vi "UHR-Fleezers Control (host) - 10.5.vi"() -> ()   [LabVIEW 2010] (continued)
          tunnel: [w3296 w3297] -> w3263
          frame False {
          }
          frame True {
            n566 = Array Subset(array=w3302, index (row)=0 ("index"), length (row)=4 ("length"), index (col)=0 ("index"), length (col)=1 ("length")) -> (w3297:T44)
          }
        }
        n567 = feedback-in #9(w3263) -> ()
        n568 = Split 1D Array(array=w3277, index=2) -> (first subarray=→"FFT 1":cluster{"f0":dbl, "df":dbl, "magnitude":dbl[]}[], second subarray=→"FFT 2":cluster{"f0":dbl, "df":dbl, "magnitude":dbl[]}[])
      }
    }
    n569 = Index Array(array=w1002, index=1) -> (element=w1010:waveform(dbl))
    n570 = case "For displaying the high resolution display (no downsampling)" shown="True" w1075 {
      tunnel: w1029 -> [_ w1535]
      frame False {
      }
      frame True {
        n571 = Index Array(array=w1535, index="High Res. Display") -> (element=w1536:waveform(dbl))
        n572 = call <vilib>:"Std Deviation and Variance.vi"("X"=w1536) -> ("mean"=w1543:dbl, "standard deviation"=w1548:dbl)  [unwired: 1 in, 1 out]
        "Mean Intensity" <- w1543
        "Sigma" <- w1548
        n573 = Subtract(x=w1536, y=w1543) -> (x-y=w1542:waveform(dbl))
        n574 = Select(t=w1542, s="Subtract mean", f=w1536) -> (s? t:f=→"1 Channel":waveform(dbl))
        n575 = Divide(x=w1548, y=w1543) -> (x/y=→"Sigma/Mean":dbl)
        n576 = feedback #10(1) -> (w1537:i32)
        n577 = Greater Or Equal?(x=w1537, y="Slow mean N ave.") -> (x >= y?=w1550:bool)
        n578 = Increment(x=w1537) -> (x+1=w1552:i32)
        n579 = Select(t=1, s=w1550, f=w1552) -> (s? t:f=w1539:i32)
        n580 = feedback-in #10(w1539) -> ()
        n581 = feedback #11() -> (w1540:waveform(dbl))  [unwired: 1 out]
        n582 = case shown="Default" w1537 {
          tunnel: [w1555 w1558] -> w1541
          tunnel: w1540 -> [w1557 _]
          tunnel: w1536 -> [w1556 w1558]
          frame Default {
            n583 = call-poly <vilib>:"Append Waveforms.vi"("waveform B"=w1556, "waveform A"=w1557) -> ("waveform out"=w1555:waveform(dbl))  [unwired: 1 in, 8 out]
          }
          frame 1 {
          }
        }
        n584 = feedback-in #11(w1541) -> ()
        n585 = case shown="True" w1550 {
          tunnel: w1541 -> [_ w1554]
          frame False {
          }
          frame True {
            n586 = call <vilib>:"Mean.vi"("X"=w1554) -> ("mean"=→"Slow mean":dbl)  [unwired: 1 out]
          }
        }
      }
    }
    n587 = case "For plotting results of scanning MCL" shown="True" w1152 {
      tunnel: w1151 -> [_ w2066]
      tunnel: w1068 -> [_ w2162]
      tunnel: w1160 -> [_ _]
      tunnel: w1029 -> [_ w2136]
      tunnel: w1004 -> [_ w2067]
      tunnel: w1003 -> [_ w2040]
      frame False {
      }
      frame True {
        w2047 = u32 0 items=["Horizontal", "Vertical", "Central", "1st Diagonal", "2nd Diagonal"] ("Type of Symmetry")
        w2075 = u32 0 items=["Horizontal", "Vertical", "Central", "1st Diagonal", "2nd Diagonal"] ("Type of Symmetry")
        w2078 = u32 0 items=["Horizontal", "Vertical", "Central", "1st Diagonal", "2nd Diagonal"] ("Type of Symmetry")
        w2107 = u32 0 items=["Horizontal", "Vertical", "Central", "1st Diagonal", "2nd Diagonal"] ("Type of Symmetry")
        n588 = Index Array(array=w2136, index=10) -> (element=w2142:waveform(dbl))
        n589 = Index Array(array=w2136, index=11) -> (element=w2139:waveform(dbl))
        n590 = local read "Cycles/step (MCL)"() -> (w2092:u64)
        n591 = Index Array(array=w2136, index="Channel") -> (element=w2138:waveform(dbl))
        n592 = Unbundle(w2040) -> ("New Image"=w2039:T2, "New Image"=w2038:T2, "New Image"=w2037:T2, "New Image"=w2036:T2)
        n593 = Unbundle By Name(w2142) -> ("Y"=w2094:dbl[])
        n594 = Unbundle By Name(w2139) -> ("Y"=w2096:dbl[])
        n595 = Unbundle By Name(w2138) -> ("Y"=w2101:dbl[])
        n596 = call "downsample 1D array - double.vi"("Ave N"=w2092, "Array In"=w2094) -> ("Array Out"=w2093:dbl[])  [unwired: 1 out]
        n597 = call "downsample 1D array - double.vi"("Ave N"=w2092, "Array In"=w2096) -> ("Array Out"=w2095:dbl[])  [unwired: 1 out]
        n598 = call "downsample 1D array - double.vi"("Ave N"=w2092, "Array In"=w2101) -> ("Array Out"=w2100:dbl[])  [unwired: 1 out]
        n599 = feedback #12(w2162) -> (w2163:dbl[])
        n600 = Build Array (concatenate)(w2163, w2162) -> (w2144:dbl[])
        n601 = feedback #13(w2067) -> (w2069:dbl[])
        n602 = Build Array (concatenate)(w2069, w2067) -> (w2068:dbl[])
        n603 = local read "Scan steps (MCL)"() -> (w2049:u64)
        n604 = Select(t=w2162, s=w2066, f=w2144) -> (s? t:f=w2148:dbl[])
        n605 = feedback-in #12(w2148) -> ()
        n606 = Select(t=w2067, s=w2066, f=w2068) -> (s? t:f=w2050:dbl[])
        n607 = feedback-in #13(w2050) -> ()
        n608 = local read "Scan lines (y)"() -> (w2035:u64)
        n609 = local read "N APD Samp/step"() -> (w2051:dbl)
        n610 = feedback #14(w2093) -> (w2150:dbl[])
        n611 = Build Array (concatenate)(w2150, w2093) -> (w2141:dbl[])
        n612 = feedback #15(w2100) -> (w2160:dbl[])
        n613 = Build Array (concatenate)(w2160, w2100) -> (w2159:dbl[])
        n614 = feedback #16(w2095) -> (w2152:dbl[])
        n615 = Build Array (concatenate)(w2152, w2095) -> (w2153:dbl[])
        n616 = Select(t=w2093, s=w2066, f=w2141) -> (s? t:f=w2097:dbl[])
        n617 = feedback-in #14(w2097) -> ()
        n618 = Select(t=w2100, s=w2066, f=w2159) -> (s? t:f=w2099:dbl[])
        n619 = feedback-in #15(w2099) -> ()
        n620 = Select(t=w2095, s=w2066, f=w2153) -> (s? t:f=w2098:dbl[])
        n621 = feedback-in #16(w2098) -> ()
        n622 = Multiply(x=w2049, y=u64 2) -> (x*y=w2034:u64)
        n623 = call "integrate 1D array interval - double.vi"("Ave N"=w2051, "Array In"=w2050) -> ("Array Out"=w2062:dbl[])  [unwired: 1 out]
        n624 = call "integrate 1D array interval - double.vi"("Ave N"=w2051, "Array In"=w2148) -> ("Array Out"=w2147:dbl[])  [unwired: 1 out]
        n625 = Array Size(array=w2062) -> (size(s)=w2063:i32)
        n626 = Array Size(array=w2147) -> (size(s)=w2149:i32)
        n627 = Multiply(x=w2035, y=w2034) -> (x*y=w2065:u64)
        n628 = Multiply(x=w2035, y=w2034) -> (x*y=w2157:u64)
        n629 = call <vilib>:"Mean.vi"("X"=w2097) -> ("mean"=w2081:dbl)  [unwired: 1 out]
        n630 = Subtract(x=w2065, y=w2063) -> (x-y=w2056:u64)
        n631 = call <vilib>:"Mean.vi"("X"=w2099) -> ("mean"=w2086:dbl)  [unwired: 1 out]
        n632 = call <vilib>:"Mean.vi"("X"=w2098) -> ("mean"=w2084:dbl)  [unwired: 1 out]
        n633 = call <vilib>:"Mean.vi"("X"=w2062) -> ("mean"=w2053:dbl)  [unwired: 1 out]
        n634 = Subtract(x=w2157, y=w2149) -> (x-y=w2091:u64)
        n635 = call <vilib>:"Mean.vi"("X"=w2147) -> ("mean"=w2088:dbl)  [unwired: 1 out]
        n636 = Initialize Array(1.0 ("element"), w2056) -> (w2052:dbl[])
        n637 = Initialize Array(1.0 ("element"), w2091) -> (w2082:dbl[])
        n638 = Multiply(x=w2052, y=w2053) -> (x*y=w2054:dbl[])
        n639 = Multiply(x=w2082, y=w2084) -> (x*y=w2085:dbl[])
        n640 = Multiply(x=w2082, y=w2086) -> (x*y=w2087:dbl[])
        n641 = Multiply(x=w2082, y=w2081) -> (x*y=w2083:dbl[])
        n642 = Multiply(x=w2082, y=w2088) -> (x*y=w2089:dbl[])
        n643 = Build Array (concatenate)(w2097, w2083) -> (w2151:dbl[])
        n644 = Build Array (concatenate)(w2099, w2087) -> (w2155:dbl[])
        n645 = Build Array (concatenate)(w2098, w2085) -> (w2154:dbl[])
        n646 = Build Array (concatenate)(w2062, w2054) -> (w2064:dbl[])
        n647 = Build Array (concatenate)(w2147, w2089) -> (w2156:dbl[])
        n648 = Reshape Array(w2151, w2035, w2034) -> (w2117:dbl[][])
        n649 = Reshape Array(w2064, w2035, w2034) -> (w2060:dbl[][])
        n650 = Reshape Array(w2155, w2035, w2034) -> (w2109:dbl[][])
        n651 = Reshape Array(w2154, w2035, w2034) -> (w2124:dbl[][])
        n652 = Reshape Array(w2156, w2035, w2034) -> (w2134:dbl[][])
        n653 = Array Subset(array=w2124, index (col)=0 ("index"), length (col)=w2049) -> (w2129:dbl[][])  [unwired: 2 in]
        n654 = Array Subset(array=w2124, index (col)=w2049) -> (w2127:dbl[][])  [unwired: 3 in]
        n655 = Array Subset(array=w2109, index (col)=0 ("index"), length (col)=w2049) -> (w2115:dbl[][])  [unwired: 2 in]
        n656 = Array Subset(array=w2109, index (col)=w2049) -> (w2113:dbl[][])  [unwired: 3 in]
        n657 = Array Subset(array=w2060, index (col)=0 ("index"), length (col)=w2049) -> (w2059:dbl[][])  [unwired: 2 in]
        n658 = Array Subset(array=w2060, index (col)=w2049) -> (w2057:dbl[][])  [unwired: 3 in]
        n659 = Array Subset(array=w2134, index (col)=0 ("index"), length (col)=w2049) -> (w2133:dbl[][])  [unwired: 2 in]
        n660 = Array Subset(array=w2134, index (col)=w2049) -> (w2131:dbl[][])  [unwired: 3 in]
        n661 = Array Subset(array=w2117, index (col)=0 ("index"), length (col)=w2049) -> (w2122:dbl[][])  [unwired: 2 in]
        n662 = Array Subset(array=w2117, index (col)=w2049) -> (w2120:dbl[][])  [unwired: 3 in]
        n663 = for {
          tunnel: w2129 -> [w2171] mode=indexing
          tunnel: [w2170] -> w2128 mode=indexing
          workers-P: _ -> [_]
          n664 = Reverse 1D Array(array=w2171) -> (reversed array=w2170:dbl[])
        }
        n665 = for {
          tunnel: w2115 -> [w2167] mode=indexing
          tunnel: [w2166] -> w2114 mode=indexing
          workers-P: _ -> [_]
          n666 = Reverse 1D Array(array=w2167) -> (reversed array=w2166:dbl[])
        }
        n667 = for {
          tunnel: w2059 -> [w2165] mode=indexing
          tunnel: [w2164] -> w2058 mode=indexing
          workers-P: _ -> [_]
          n668 = Reverse 1D Array(array=w2165) -> (reversed array=w2164:dbl[])
        }
        n669 = for {
          tunnel: w2133 -> [w2173] mode=indexing
          tunnel: [w2172] -> w2132 mode=indexing
          workers-P: _ -> [_]
          n670 = Reverse 1D Array(array=w2173) -> (reversed array=w2172:dbl[])
        }
        n671 = for {
          tunnel: w2122 -> [w2169] mode=indexing
          tunnel: [w2168] -> w2121 mode=indexing
          workers-P: _ -> [_]
          n672 = Reverse 1D Array(array=w2169) -> (reversed array=w2168:dbl[])
        }
        n673 = Index Array(array=w2134, index (row)=0) -> (element=→"Waveform Graph":dbl[])  [unwired: 1 in]
        n674 = Add(x=w2128, y=w2127) -> (x+y=w2126:dbl[][])
        n675 = Add(x=w2114, y=w2113) -> (x+y=w2112:dbl[][])
        n676 = Add(x=w2058, y=w2057) -> (x+y=w2042:dbl[][])
        n677 = Add(x=w2132, y=w2131) -> (x+y=w2106:dbl[][])
        n678 = Add(x=w2121, y=w2120) -> (x+y=w2119:dbl[][])
        n679 = Divide(x=w2112, y=2) -> (x/y=w2110:dbl[][])
        n680 = Divide(x=w2126, y=2) -> (x/y=w2071:dbl[][])
        n681 = Divide(x=w2119, y=2) -> (x/y=w2073:dbl[][])
        n682 = To Single Precision Float(number=w2106) -> (single precision float=w2105:sgl[][])
        n683 = Transpose 2D Array(2D array=w2110) -> (transposed array=→"Data map":dbl[][])
        n684 = To Single Precision Float(number=w2042) -> (single precision float=w2046:sgl[][])
        n685 = To Single Precision Float(number=w2071) -> (single precision float=w2077:sgl[][])
        n686 = To Single Precision Float(number=w2073) -> (single precision float=w2074:sgl[][])
        n687 = call "IMAQ ArrayToImage"("Image Pixels (Float)"=w2105, "Image"=w2039) -> ("Image Out"=w2108:T2)  [unwired: 8 in, 1 out]
        n688 = call "IMAQ ArrayToImage"("Image Pixels (Float)"=w2046, "Image"=w2038) -> ("Image Out"=w2048:T2)  [unwired: 8 in, 1 out]
        n689 = call "IMAQ ArrayToImage"("Image Pixels (Float)"=w2077, "Image"=w2037) -> ("Image Out"=w2079:T2)  [unwired: 8 in, 1 out]
        n690 = call "IMAQ ArrayToImage"("Image Pixels (Float)"=w2074, "Image"=w2036) -> ("Image Out"=w2076:T2)  [unwired: 8 in, 1 out]
        n691 = call "IMAQ Symmetry"("Type of Symmetry"=w2107, "Image Src"=w2108) -> ("Image Dst Out"=w2103:T2)  [unwired: 3 in, 1 out]
        n692 = call "IMAQ Symmetry"("Type of Symmetry"=w2047, "Image Src"=w2048) -> ("Image Dst Out"=w2044:T2)  [unwired: 3 in, 1 out]
        n693 = call "IMAQ Symmetry"("Type of Symmetry"=w2078, "Image Src"=w2079) -> ("Image Dst Out"=→"Detection Laser X":T2)  [unwired: 3 in, 1 out]
        n694 = call "IMAQ Symmetry"("Type of Symmetry"=w2075, "Image Src"=w2076) -> ("Image Dst Out"=→"Detection Laser Y":T2)  [unwired: 3 in, 1 out]
        n695 = call "IMAQ Set Simple Calibration"("Calibration Axis Info"=T31 {"Origin Pixel"={"X"=0.0, "Y"=0.0}, "Angle Relative to Horizontal (deg)"=0.0, "Axis Reference"=0}, "Grid Descriptor"=T32 {"X Step"=0.3, "Y Step"=0.3, "Unit"=enum."Undefined"}, "Image"=w2103) -> ("Calibrated Image"=→"APD 1":T2)  [unwired: 7 in, 1 out]
        n696 = call "IMAQ Set Simple Calibration"("Calibration Axis Info"=T31 {"Origin Pixel"={"X"=0.0, "Y"=0.0}, "Angle Relative to Horizontal (deg)"=0.0, "Axis Reference"=0}, "Grid Descriptor"=T32 {"X Step"=0.3, "Y Step"=0.3, "Unit"=enum."Undefined"}, "Image"=w2044) -> ("Calibrated Image"=→"APD 2":T2)  [unwired: 7 in, 1 out]
      }
    }
    n697 = Subtract(x=w1010, y="APD 2 Offset") -> (x-y=w1007:waveform(dbl))
    n698 = Subtract(x=w1012, y="APD 1 Offset") -> (x-y=w1008:waveform(dbl))
    n699 = Index Array(array=w1027, index=3) -> (element=w1096:waveform(dbl))
    n700 = Index Array(array=w1027, index=6) -> (element=w1093:waveform(dbl))
    n701 = Build Array(w1008, w1007) -> (→"APD Chart":waveform(dbl)[])
    n702 = Array Size(array=w1085) -> (size(s)=w1140:i32)
    n703 = call <vilib>:"Std Deviation and Variance.vi"("X"=w1020) -> ("standard deviation"=w1019:dbl)  [unwired: 1 in, 2 out]
    n704 = Add Array Elements(numeric array=w1020) -> (sum=w1022:u32)
    n705 = Add Array Elements(numeric array=w1085) -> (sum=w1150:u32)
    n706 = call <vilib>:"Std Deviation and Variance.vi"("X"=w1085) -> ("standard deviation"=w1084:dbl)  [unwired: 1 in, 2 out]
    n707 = Divide(x="T1 offset_x (mV)", y=1000.0) -> (x/y=w1097:dbl)
    n708 = Divide(x=w1019, y=w1018) -> (x/y=w1015:dbl)
    "Rate sigma (Hz) 2" <- w1015
    n709 = Multiply(x=w1018, y=w1140) -> (x*y=w1021:dbl)
    "Int. Time (s)" <- w1021
    n710 = Divide(x=w1022, y=w1021) -> (x/y=w1016:dbl)
    "APD 2 Rate (Hz)" <- w1016
    n711 = Divide(x=w1150, y=w1021) -> (x/y=w1082:dbl)
    "APD 1 Rate (Hz)" <- w1082
    n712 = Divide(x=w1084, y=w1018) -> (x/y=w1083:dbl)
    "Rate sigma (Hz)" <- w1083
    n713 = Divide(x=w1015, y=w1016) -> (x/y=→"Sigma/Mean 2":dbl)
    n714 = Divide(x=w1083, y=w1082) -> (x/y=→"Sigma/Mean":dbl)
    n715 = Divide(x="T2 offset_x (mV)", y=1000.0) -> (x/y=w1095:dbl)
    n716 = case shown="2" "Calibration" {
      tunnel: "T1 alpha_x (nm/V)" -> [_ w2002 w2023]
      tunnel: "T1 kappa_x (pN/nm)" -> [_ _ w2013]
      tunnel: "T2 alpha_x (nm/V)" -> [_ w2001 w2021]
      tunnel: "T2 kappa_x (pN/nm)" -> [_ _ w2014]
      tunnel: w1096 -> [w1984 w1999 w2019]
      tunnel: w1093 -> [w1983 w1997 w2017]
      tunnel: [w1984 w1996 w2016] -> w1126
      tunnel: [w1983 w1995 w2015] -> w1125
      tunnel: ["T1 X (V)" ("Label.Text") "T1 X (nm)" ("Label.Text") "T1 X (pN)" ("Label.Text")] -> w1114
      tunnel: ["T2 X (V)" ("Label.Text") "T2 X (nm)" ("Label.Text") "T2 X (pN)" ("Label.Text")] -> w1113
      tunnel: ["Position (V)" ("Label.Text") "Position (nm)" ("Label.Text") "Force (pN)" ("Label.Text")] -> w1115
      tunnel: w1095 -> [_ w1987 w2006]
      tunnel: w1097 -> [_ w1990 w2008]
      tunnel: ["Mean (V)" ("Label.Text") "Mean (nm)" ("Label.Text") "Mean (pN)" ("Label.Text")] -> w1110
      tunnel: ["Difference (V)" ("Label.Text") "Difference (nm)" ("Label.Text") "Difference (pN)" ("Label.Text")] -> w1035
      frame 0, Default {
      }
      frame 1 {
        # "position"
        n717 = Unbundle By Name(w1999) -> ("Y"=w2003:dbl[])
        n718 = Unbundle By Name(w1997) -> ("Y"=w1988:dbl[])
        n719 = Subtract(x=w2003, y=w1990) -> (x-y=w1991:dbl[])
        n720 = Subtract(x=w1988, y=w1987) -> (x-y=w1989:dbl[])
        n721 = Multiply(x=w1989, y=w2001) -> (x*y=w1998:dbl[])
        n722 = Multiply(x=w2002, y=w1991) -> (x*y=w2000:dbl[])
        n723 = Bundle By Name(cluster=w1997, "Y"=w1998) -> (w1995:waveform(dbl))
        n724 = Bundle By Name(cluster=w1999, "Y"=w2000) -> (w1996:waveform(dbl))
      }
      frame 2 {
        # "force"
        n725 = Unbundle By Name(w2019) -> ("Y"=w2024:dbl[])
        n726 = Unbundle By Name(w2017) -> ("Y"=w2022:dbl[])
        n727 = Subtract(x=w2022, y=w2006) -> (x-y=w2007:dbl[])
        n728 = Subtract(x=w2024, y=w2008) -> (x-y=w2009:dbl[])
        n729 = Compound Arithmetic op=MULTIPLY(w2007, w2021, w2014) -> (w2018:dbl[])
        n730 = Compound Arithmetic op=MULTIPLY(w2013, w2023, w2009) -> (w2020:dbl[])
        n731 = Bundle By Name(cluster=w2017, "Y"=w2018) -> (w2015:waveform(dbl))
        n732 = Bundle By Name(cluster=w2019, "Y"=w2020) -> (w2016:waveform(dbl))
      }
    }
    n733 = feedback-in #17("Calibration") -> ()
    n734 = feedback #17(u16 1 ("Calibration")) -> (w1117:u16)
    n735 = Not Equal?(x=w1117, y="Calibration") -> (x != y?=w1073:bool)
    n736 = Unbundle By Name(w1096) -> ("Y"=w1099:dbl[])
    n737 = Unbundle By Name(w1093) -> ("Y"=w1102:dbl[])
    n738 = Subtract(x=w1099, y=w1097) -> (x-y=w1100:dbl[])
    n739 = Subtract(x=w1102, y=w1095) -> (x-y=w1101:dbl[])
    n740 = Multiply(x=w1101, y="T2 alpha_x (nm/V)") -> (x*y=w1092:dbl[])
    n741 = Multiply(x="T1 alpha_x (nm/V)", y=w1100) -> (x*y=w1091:dbl[])
    n742 = Multiply(x=w1125, y=-1.0) -> (x*y=w1104:waveform(dbl))
    n743 = case shown="True" "Read Lateness and Rel Phase" {
      tunnel: w926 -> [w1559 w1581]
      tunnel: w925 -> [w1560 w1580]
      tunnel: [w1559 w1579] -> w1088
      tunnel: [w1560 w1578] -> w1087
      frame False {
      }
      frame True {
        n744 = xnode "Read/Write Control"("FPGA VI Reference In"=w1581, "error in"=w1580) -> ("FPGA VI Reference Out"=w1579:T20, "error out"=w1578:errorcluster, "GI Relative phase"=→"GI relative phase":i16, "Relative phase"=→"Relative phase (AI1)":i16, "AI Late Counter"=→"Late Counter (AI1)":u16, "GI Late Counter"=→"GI Late Counter":u16, "MCL Late Counter"=→"MCL Late Counter":u16, "MCL Relative Phase"=→"Relative Phase (MCL)":i16, "APD Acq Relative Phase"=→"APD Acq Relative Phase":i16, "APD 1 Gate Relative Phase"=→"APD 1 Gate Relative Phase":i16, "APD 2 Gate Relative Phase"=→"APD 2 Gate Relative Phase":i16, "APD Acq Late Counter"=→"APD Acq Late Counter":u16, "APD 1 Gate Late Counter"=→"APD 1 Gate Late Counter":u16, "APD 2 Gate Late Counter"=→"APD 2 Gate Late Counter":u16, "Green FB Relative Phase"=→"Relative phase (Green FB)":i16, "GI Relative phase 2"=→"GI relative phase 2":i16, "GI Late Counter 2"=→"GI Late Counter 2":u16, "Trap Pos FIFO Timeout"=→"Trap Pos FIFO Timeout":u16, "Trap AI FIFO Timeout"=→"Trap AI FIFO Timeout":u16)
      }
    }
    n745 = Subtract(x=w1092, y=w1091) -> (x-y=w1090:dbl[])
    n746 = Unbundle By Name(w1125) -> ("Y"=w1060:dbl[])
    n747 = Unbundle By Name(w1126) -> ("Y"=w1061:dbl[])
    n748 = Build Array(w1126, w1104) -> (→"Force":waveform(dbl)[])
    n749 = Subtract(x=w1090, y="Offset (nm)") -> (x-y=w1058:dbl[])
    n750 = call <vilib>:"Mean.vi"("X"=w1060) -> ("mean"=w1039:dbl)  [unwired: 1 out]
    "T2 X" <- w1039
    n751 = Absolute Value(x=w1061) -> (abs(x)=w1062:dbl[])
    n752 = Absolute Value(x=w1060) -> (abs(x)=w1063:dbl[])
    n753 = call <vilib>:"Mean.vi"("X"=w1061) -> ("mean"=w1040:dbl)  [unwired: 1 out]
    "T1 X" <- w1040
    n754 = Add(x=w1062, y=w1063) -> (x+y=w1064:dbl[])
    n755 = Bundle By Name(cluster=w1096, "Y"=w1058) -> (w1026:waveform(dbl))
    "Bead Separation" <- w1026
    n756 = Divide(x=w1064, y=2.0) -> (x/y=→"Vec Mean of T1 T2":dbl[])
    n757 = case shown="True" w1073 {
      tunnel: w1115 -> [_ w1977]
      tunnel: w1114 -> [_ w1976]
      tunnel: w1113 -> [_ w1975]
      tunnel: w1110 -> [_ w1974]
      tunnel: w1035 -> [_ w1973]
      frame False {
      }
      frame True {
        n758 = property on="Force" class="WFChart (strict)"("YScale.NameLbl.Text"=w1977) -> ()  [unwired: 2 in, 2 out]
        n759 = property on="T2 X" class="DigNum (strict)"("Caption.Text"=w1975) -> ()  [unwired: 2 in, 2 out]
        n760 = property on="T1 X" class="DigNum (strict)"("Caption.Text"=w1976) -> ()  [unwired: 2 in, 2 out]
        n761 = property on="Mean" class="DigNum (strict)"("Caption.Text"=w1974) -> ()  [unwired: 2 in, 2 out]
        n762 = property on="Difference" class="DigNum (strict)"("Caption.Text"=w1973) -> ()  [unwired: 2 in, 2 out]
      }
    }
    n763 = local read "Tether"() -> (w1067:bool)
    n764 = Absolute Value(x=w1040) -> (abs(x)=w1037:dbl)
    n765 = Absolute Value(x=w1039) -> (abs(x)=w1036:dbl)
    n766 = Add(x=w1037, y=w1036) -> (x+y=w1112:dbl)
    n767 = Subtract(x=w1037, y=w1036) -> (x-y=→"Difference":dbl)
    n768 = feedback #18(w1058) -> (w1057:dbl[])
    n769 = Divide(x=w1112, y=2.0) -> (x/y=w1066:dbl)
    "Mean" <- w1066
    n770 = case shown="True" w1067 {
      tunnel: w1066 -> [_ w1518]
      frame False {
      }
      frame True {
        n771 = Greater?(x="Lost Tether Alarm Threshold (pN)", y=w1518) -> (0:w1516:bool)
        n772 = case shown="True" w1516 {
          frame False {
          }
          frame True {
            n773 = flat-sequence {
              frame #0 {
                # "stop only if saving"
                n774 = local read "Saving..."() -> (w1531:bool)
                n775 = And(x=w1531, y="TA Cancel Save?") -> (x .and. y?=w1530:bool)
                n776 = local write "Stop Saving"(w1530) -> ()
              }
              frame #1 {
                n777 = case shown="True" "TA Green Off?" {
                  frame False {
                  }
                  frame True {
                    w1534 = FALSE ("Fl. Triggered...")
                    n778 = local write "Fl. Triggered..."(w1534) -> ()
                    n779 = property on="Green Laser ON/Interlacing" class="Bool (strict)"("Val(Sgnl)"=w1534) -> ()  [unwired: 2 in, 2 out]
                  }
                }
              }
            }
            n780 = local read "Time tether formed"() -> (w1525:timestamp)
            n781 = Get Date/Time In Seconds() -> (seconds since 1Jan1904=w1526:timestamp)
            n782 = Subtract(x=w1526, y=w1525) -> (x-y=w1524:dbl)
            n783 = Number To Decimal String(number=w1524) -> (decimal integer string=w1521:string)  [unwired: 1 out]
            n784 = local read "Messages"() -> (w1528:string)
            n785 = call <vilib>:"Beep.vi"() -> ()  [unwired: 3 in, 9 out]
            n786 = Concatenate Strings("Lost tether (" ("Message to add"), w1521, " s)." ("string")) -> (w1523:string)
            n787 = local write "Tether"(FALSE ("Tether")) -> ()
            n788 = call "Update messages.vi"("Message to add"=w1523, "Old message string"=w1528) -> ("New message string"=w1527:string)
            n789 = local write "Messages"(w1527) -> ()
            n790 = property on="Trap Pos. FB ON" class="Bool (strict)"("Val(Sgnl)"=FALSE ("Value (Signaling)")) -> ()  [unwired: 2 in, 2 out]
          }
        }
      }
    }
    n791 = Build Array (concatenate)(w1058, w1057) -> (w1056:dbl[])
    n792 = Split 1D Array(array=w1056, index=w938) -> (first subarray=w1052:dbl[])  [unwired: 1 out]
    n793 = feedback-in #18(w1052) -> ()
    n794 = call <vilib>:"Mean.vi"("X"=w1052) -> ("mean"=w1051:dbl)  [unwired: 1 out]
    "Bead Mean (nm)" <- w1051
    n795 = Subtract(x=w1052, y=w1051) -> (x-y=w1050:dbl[])
    n796 = Square(x=w1050) -> (x^2=w1049:dbl[])
    n797 = call <vilib>:"Mean.vi"("X"=w1049) -> ("mean"=w1048:dbl)  [unwired: 1 out]
    n798 = Square Root(x=w1048) -> (sqrt(x)=w1047:dbl)
    n799 = Multiply(x=10.0, y=w1047) -> (x*y=→"RMS (Ang)":dbl)
    n800 = xnode "Read/Write Control"("FPGA VI Reference In"=w1088, "error in"=w1087) -> ("FPGA VI Reference Out"=w1206:T20, "error out"=w1200:errorcluster, "AI2 Y Sum Set 1"=w1196:i16, "AI2 Y Sum Set 2"=w1195:i16, "AI1 X Set 1"=w972:fxp<+/-,16,1>, "AI1 X Set 2"=w971:fxp<+/-,16,1>, "Trap Pos FB Int Signal"=→"Trap Pos FB Int Signal":fxp<+/-,24,9>, "Trap Pos FB Int-Norm Signal"=→"Trap Pos FB Int-Norm Signal":fxp<+/-,16,1>, "Trap Pos FB Action"=w965:i64, "Scanning"=→"AOD Scanning":bool, "Scan I"=→"AOD Scan I":u64, "Scanning MCL"=w1198:bool, "Scan I (MCL)"=→"MCL Scan I":u64, "Green FB Signals"=w1135:T36)  [unwired: 1 out]
    "MCL Scanning" <- w1198
    "Trap Pos FB Action" <- w965
    n801 = local read "AI2 (V)"() -> (w1197:cluster{"Set 1":dbl, "Set 2":dbl})
    n802 = Bundle By Name(cluster=w1197, "Set 1"=w1196, "Set 2"=w1195) -> (w1193:cluster{"Set 1":dbl, "Set 2":dbl})
    n803 = Divide(x=w965, y=327.67) -> (x/y=→"Action (%)":dbl)
    n804 = local read "Trap X (AI1)"() -> (w985:T11)
    n805 = Divide(x=w1193, y=3276.7) -> (x/y=w1192:cluster{"Set 1":dbl, "Set 2":dbl})
    n806 = local write "AI2 (V)"(w1192) -> ()
    n807 = Bundle(cluster=w985, "Trap 1"=w972, "Trap 2"=w971) -> (→"Trap X (AI1)":T11)
    n808 = Divide(x=w1135, y=3276.7) -> (x/y=w1131:T45)
    n809 = Unbundle By Name(w1131) -> ("Green FB Ch 0"=w1134:dbl, "Green FB Ch 1"=w1133:dbl, "Green FB Ch 2"=w1132:dbl)
    n810 = Divide(x=w1134, y=w1132) -> (x/y=w1130:dbl)
    n811 = Divide(x=w1133, y=w1132) -> (x/y=w1129:dbl)
    n812 = flat-sequence "To save data" {
      tunnel: [w3770] -> w1217
      tunnel: [w3771] -> w1216
      tunnel: w1166 -> [w3764]
      tunnel: w1054 -> [w3768]
      tunnel: ["Save Calibration"] -> w1189
      tunnel: w1186 -> [w3767]
      tunnel: [w3760] -> w1185
      tunnel: [w3757] -> w1184
      tunnel: [w3754] -> w1183
      tunnel: w1165 -> [w3756]
      tunnel: w1071 -> [w3750]
      tunnel: [w3750] -> w1070
      tunnel: ["Start Saving"] -> w1028
      tunnel: [w3744] -> w954
      tunnel: [w3743] -> w953
      tunnel: w1217 -> [w4005]
      tunnel: w1216 -> [w4004]
      tunnel: w955 -> [w4003]
      tunnel: w1189 -> [w4002]
      tunnel: w1185 -> [w4000]
      tunnel: w1184 -> [w3999]
      tunnel: w1183 -> [w3998]
      tunnel: w1041 -> [w3997]
      tunnel: w1080 -> [w3996]
      tunnel: w1070 -> [w3995]
      tunnel: w1028 -> [w3994]
      tunnel: w1026 -> [w3993]
      tunnel: w1002 -> [w3992]
      tunnel: w954 -> [w3991]
      tunnel: w953 -> [w3990]
      tunnel: w952 -> [w3989]
      frame #0 {
        n813 = Or(x="Save N Sets", y="Start Saving") -> (x .or. y?=w3751:bool)
        n814 = To Double Precision Float(number=w3767) -> (double precision float=w3761:dbl)
        n815 = Build Array(w3751, "Save Calibration", w3764, w3756) -> (w3766:bool[])
        n816 = Compound Arithmetic op=OR("Save Calibration", w3764, w3751, w3756) -> (w3769:bool)
        n817 = Boolean Array To Number(Boolean array=w3766) -> (number=w3763:u32)
        n818 = feedback #19(FALSE ("Save APD Data\nwith Trap Data")) -> (w3745:bool)
        n819 = feedback #20(refnum<k0> refnum) -> (w3772:refnum<file>)
        n820 = feedback #21(refnum<k0> refnum) -> (w3747:refnum<file>)
        n821 = feedback #22(FALSE ("Save APD Data\nwith Trap Data")) -> (w3755:bool)
        n822 = feedback #23(refnum<k0> refnum) -> (w3758:refnum<file>)
        n823 = feedback #24(0) -> (w3774:i32)
        n824 = feedback #25() -> (w3762:u32)  [unwired: 1 out]
        n825 = case shown="False" w3769 {
          tunnel: [w3781 1] -> w3770
          tunnel: w3774 -> [w3783 _]
          tunnel: [w3782 w3801] -> w3771
          tunnel: w3772 -> [w3782 _]
          tunnel: w3768 -> [_ w3821]
          tunnel: w3761 -> [_ w3819]
          tunnel: w3763 -> [_ w3822]
          tunnel: [w3780 w3800] -> w3760
          tunnel: w3762 -> [w3780 _]
          tunnel: [w3779 w3798] -> w3757
          tunnel: w3758 -> [w3779 _]
          tunnel: [w3778 w3797] -> w3754
          tunnel: w3755 -> [w3778 _]
          tunnel: "Start Saving" -> [_ w3795]
          tunnel: w3750 -> [_ w3794]
          tunnel: [w3777 w3785] -> w3743
          tunnel: w3747 -> [w3777 _]
          tunnel: [w3776 w3784] -> w3744
          tunnel: w3745 -> [w3776 _]
          frame False {
            n826 = Increment(x=w3783) -> (x+1=w3781:i32)
          }
          frame True {
            w3791 = FALSE ("Start Saving")
            w3796 = 9.0  # File Version
            w3804 = FALSE ("prepend array or string size? (T)")
            w3802 = T38."big-endian, network order" ("byte order (0:big-endian, network order)")
            n827 = local read "BD 1 Frequency 1 (MHz)"() -> (w3818:dbl)
            n828 = local read "BD 2 Frequency 1 (MHz)"() -> (w3817:dbl)
            n829 = local read "BD 1 Frequency 2 (MHz)"() -> (w3816:dbl)
            n830 = local read "BD 2 Frequency 2 (MHz)"() -> (w3815:dbl)
            n831 = local read "BD 1 Frequency 3 (MHz)"() -> (w3814:dbl)
            n832 = local read "BD 2 Frequency 3 (MHz)"() -> (w3813:dbl)
            n833 = Array Size(array=w3794) -> (size(s)=w3793:i32)
            n834 = To Double Precision Float(number=w3793) -> (double precision float=w3792:dbl)
            n835 = local write "Save Calibration"(w3791) -> ()
            n836 = local write "Start Saving"(w3791) -> ()
            n837 = Build Array("Save APD Data\nwith Trap Data", "Save Trap Pos. Data") -> (w3788:bool[])
            n838 = Boolean Array To Number(Boolean array=w3788) -> (number=w3787:u32)
            n839 = Build Array(w3818, w3817, w3816, w3815, w3814, w3813) -> (w3812:dbl[])
            n840 = case shown="1, Default" w3822 {
              tunnel: w3821 -> [w3893 w3913 w3929 w3967]
              tunnel: w3792 -> [w3898 w3920 w3949 w3986]
              tunnel: w3819 -> [w3897 w3919 w3948 w3985]
              tunnel: [w3894 w3915 w3940 w3977] -> w3810
              tunnel: [w3885 "Cal sets to save" w3930 w3968] -> w3800
              tunnel: w3812 -> [w3895 w3916 w3942 w3979]
              tunnel: "Save APD Data\nwith Trap Data" -> [w3892 _ w3926 w3965]
              tunnel: [w3892 w3907 w3926 w3965] -> w3797
              tunnel: w3796 -> [w3888 w3908 w3924 w3963]
              tunnel: w3795 -> [w3887 _ _ _]
              tunnel: [w3878 w3907 w3923 w3953] -> w3784
              tunnel: "Save Trap Pos. Data" -> [w3878 _ w3923 w3953]
              tunnel: w3787 -> [w3877 _ w3922 w3952]
              frame 1, Default {
                # "timeseries"
                n841 = case shown="True" "Profile" {
                  tunnel: [w3901 w3904] -> w3882
                  tunnel: [w3901 w3903] -> w3881
                  tunnel: [w3901 w3902] -> w3880
                  tunnel: [w3901 w3906] -> w3879
                  frame False {
                    w3901 = 0.0 ("f")
                  }
                  frame True {
                    n842 = local read "Current Position"() -> (w3905:dbl[])
                    n843 = local read "Y change (mm)"() -> (w3906:dbl)
                    n844 = call "subVI_explode3array.vi"("Array"=w3905) -> ("x"=w3904:dbl, "y"=w3903:dbl, "z"=w3902:dbl)  [unwired: 12 in]
                  }
                }
                n845 = local read "Save ave N"() -> (w3900:dbl)
                n846 = Multiply(x=w3900, y=w3893) -> (x*y=w3899:dbl)
                n847 = To Double Precision Float(number=w3877) -> (double precision float=w3891:dbl)
                n848 = Build Array(w3888, w3893, w3899, w3898, w3897, 0.0 ("f")) -> (w3896:dbl[])
                n849 = Build Array(w3891, w3882, w3881, w3880, w3879) -> (w3889:dbl[])
                n850 = Select(t=u32 4000000000, s=w3887, f="N sets to save") -> (s? t:f=w3885:u32)
                n851 = Build Array (concatenate)(w3896, w3895, w3889) -> (w3894:dbl[])
              }
              frame 2 {
                w3910 = 0.0 ("f")
                w3907 = FALSE ("Save APD Data\nwith Trap Data")
                # "calibration"
                n852 = Boolean To (0,1)(Boolean=w3907) -> (0, 1=w3912:i16)
                n853 = To Double Precision Float(number=w3912) -> (double precision float=w3911:dbl)
                n854 = Build Array(w3911, w3910, w3910, w3910, w3910) -> (w3909:dbl[])
                n855 = Build Array(w3908, w3913, w3913, w3920, w3919, 1.0 ("t")) -> (w3917:dbl[])
                n856 = Build Array (concatenate)(w3917, w3916, w3909) -> (w3915:dbl[])
                "Calibrating Trap..." <- TRUE ("Calibrating...")
              }
              frame 4 {
                w3927 = 0.0 ("f")
                # "scan dir (x/y = 0/1)"
                # "cycles/step"
                # "n scans (f/b)"
                # "steps"
                # "freq. range"
                # "AOD raster scan"
                n857 = local read "Number of F/B Scans (AOD)"() -> (w3934:u16)
                n858 = local read "Cycles/step (AOD)"() -> (w3936:u64)
                n859 = local read "Scan Range (MHz)"() -> (w3939:dbl)
                n860 = local read "Scan steps (AOD)"() -> (w3938:u64)
                n861 = local read "Scan BD"() -> (w3946:bool)
                n862 = local read "Save ave N"() -> (w3951:dbl)
                n863 = Boolean To (0,1)(Boolean=w3946) -> (0, 1=w3945:i16)
                n864 = To Double Precision Float(number=w3934) -> (double precision float=w3933:dbl)
                n865 = To Double Precision Float(number=w3938) -> (double precision float=w3937:dbl)
                n866 = To Double Precision Float(number=w3936) -> (double precision float=w3935:dbl)
                n867 = To Double Precision Float(number=w3945) -> (double precision float=w3944:dbl)
                n868 = Multiply(x=w3951, y=w3929) -> (x*y=w3950:dbl)
                n869 = To Double Precision Float(number=w3922) -> (double precision float=w3928:dbl)
                n870 = Build Array(w3928, w3927, w3927, w3927, w3927) -> (w3925:dbl[])
                n871 = local read "N sets should be saved"() -> (w3931:dbl)
                n872 = Build Array(w3944, w3939, w3937, w3935, w3933) -> (w3941:dbl[])
                n873 = Build Array(w3924, w3929, w3950, w3949, w3948, 2.0 ("t")) -> (w3943:dbl[])
                n874 = Round Toward +Infinity(x=w3931) -> (ceil(x): smallest int >= x=w3932:dbl)
                n875 = Build Array (concatenate)(w3943, w3942, w3925, w3941) -> (w3940:dbl[])
                n876 = To Unsigned Long Integer(number=w3932) -> (unsigned 32bit integer=w3930:u32)
              }
              frame 8 {
                w3960 = 0.0 ("f")
                # "MCL raster scan"
                n877 = local read "Number of scans (MCL)"() -> (w3955:u64)
                n878 = local read "Scan lines (y)"() -> (w3954:u64)
                n879 = local read "2D or 1D Scan"() -> (w3957:bool)
                n880 = local read "Scan Range (V)\n(of steps)"() -> (w3976:dbl)
                n881 = local read "Fast Scan Dir"() -> (w3983:bool)
                n882 = local read "Cycles/step (MCL)"() -> (w3973:u64)
                n883 = local read "Scan steps (MCL)"() -> (w3975:u64)
                n884 = Select(t=w3954, s=w3957, f=w3955) -> (s? t:f=w3956:u64)
                n885 = Boolean To (0,1)(Boolean=w3957) -> (0, 1=w3959:i16)
                n886 = local read "Save ave N"() -> (w3988:dbl)
                n887 = local read "Initial X"() -> (w3962:dbl)
                n888 = local read "Initial Y"() -> (w3961:dbl)
                n889 = To Double Precision Float(number=w3959) -> (double precision float=w3958:dbl)
                n890 = Boolean To (0,1)(Boolean=w3983) -> (0, 1=w3982:i16)
                n891 = To Double Precision Float(number=w3956) -> (double precision float=w3971:dbl)
                n892 = To Double Precision Float(number=w3975) -> (double precision float=w3974:dbl)
                n893 = To Double Precision Float(number=w3973) -> (double precision float=w3972:dbl)
                n894 = To Double Precision Float(number=w3982) -> (double precision float=w3981:dbl)
                n895 = Multiply(x=w3988, y=w3967) -> (x*y=w3987:dbl)
                n896 = To Double Precision Float(number=w3952) -> (double precision float=w3966:dbl)
                n897 = local read "N sets should be saved (MCL)"() -> (w3969:dbl)
                n898 = Build Array(w3966, w3958, w3960, w3960, w3960) -> (w3964:dbl[])
                n899 = Build Array(w3981, w3976, w3974, w3972, w3971, w3962, w3961) -> (w3978:dbl[])
                n900 = Build Array(w3963, w3967, w3987, w3986, w3985, 3.0 ("t")) -> (w3980:dbl[])
                n901 = Round Toward +Infinity(x=w3969) -> (ceil(x): smallest int >= x=w3970:dbl)
                n902 = Build Array (concatenate)(w3980, w3979, w3964, w3978) -> (w3977:dbl[])
                n903 = To Unsigned Long Integer(number=w3970) -> (unsigned 32bit integer=w3968:u32)
              }
            }
            n904 = local read "Index"() -> (w3827:dbl)
            n905 = call "Create new save file.vi"("Insert"="", "Ext"=".dat", "Index In"=w3827) -> ("Path Out"=w3786:path, "Index Out"=w3799:dbl)
            n906 = local write "Save file name"(w3786) -> ()
            n907 = local write "Index"(w3799) -> ()
            n908 = local write "Save index"(w3799) -> ()
            n909 = Array Size(array=w3810) -> (size(s)=w3811:i32)
            n910 = Open/Create/Replace File(file path (use dialog)=w3786, operation (0:open)=T37."create", access (0:read/write)=enum16{"read/write", "read-only", "write-only"}."write-only") -> (refnum out=w3824:refnum<file>)  [unwired: 1 in, 4 out]
            n911 = local write "Saving..."(TRUE ("Saving...")) -> ()
            n912 = To Double Precision Float(number=w3811) -> (double precision float=w3809:dbl)
            n913 = String Length(string="Comment (data description)") -> (length=w3807:i32)
            n914 = To Double Precision Float(number=w3807) -> (double precision float=w3806:dbl)
            n915 = Deny Access(7:w3824) -> (3:w3823:refnum<file>)  [unwired: 1 in, 2 out]
            n916 = Build Array (concatenate)(w3809, w3810, w3806) -> (w3808:dbl[])
            n917 = case "If fluorescence data to be saved" shown="True" w3797 {
              tunnel: w3786 -> [_ w3876]
              tunnel: [refnum<k0> refnum w3856] -> w3798
              frame False {
              }
              frame True {
                w3855 = 0.0
                n918 = local read "APD Integration Time (s)"() -> (w3861:dbl)
                n919 = local read "N APD Samp/step"() -> (w3854:dbl)
                n920 = Path To String(path=w3876) -> (string=w3875:string)
                n921 = String Length(string=w3875) -> (length=w3874:i32)
                n922 = Subtract(x=w3874, y=4) -> (x-y=w3872:i32)
                n923 = String Subset(string=w3875, length (rest)=w3872) -> (substring=w3871:string)  [unwired: 1 out]
                n924 = Build Array(w3861, w3854, w3855, w3855, w3855, w3855, w3855, w3855) -> (w3858:dbl[])
                n925 = Concatenate Strings(w3871, "_fl.dat" ("string")) -> (w3869:string)
                n926 = Array Size(array=w3858) -> (size(s)=w3860:i32)
                n927 = String To Path(string=w3869) -> (path=w3865:path)
                n928 = Open/Create/Replace File(file path (use dialog)=w3865, operation (0:open)=T37."create", access (0:read/write)=enum16{"read/write", "read-only", "write-only"}."write-only") -> (refnum out=w3866:refnum<file>)  [unwired: 1 in, 4 out]
                n929 = Deny Access(7:w3866) -> (3:w3862:refnum<file>)  [unwired: 1 in, 2 out]
                n930 = To Double Precision Float(number=w3860) -> (double precision float=w3859:dbl)
                n931 = Build Array (concatenate)(w3859, w3858) -> (w3857:dbl[])
                n932 = Write to Binary File(file (use dialog)=w3862, data=w3857, 5:FALSE ("prepend array or string size? (T)"), 9:T38."big-endian, network order" ("byte order (0:big-endian, network order)")) -> (refnum out=w3856:refnum<file>)  [unwired: 1 in, 3 out]
              }
            }
            n933 = case shown="True" w3784 {
              tunnel: w3786 -> [_ w3838]
              tunnel: [refnum<k0> refnum w3837] -> w3785
              frame False {
              }
              frame True {
                w3833 = 0.0 ("element")
                n934 = Path To String(path=w3838) -> (string=w3852:string)
                n935 = Build Array(w3833, w3833, w3833, w3833, w3833, w3833, w3833, w3833) -> (w3834:dbl[])
                n936 = String Length(string=w3852) -> (length=w3851:i32)
                n937 = Subtract(x=w3851, y=4) -> (x-y=w3849:i32)
                n938 = Array Size(array=w3834) -> (size(s)=w3836:i32)
                n939 = String Subset(string=w3852, length (rest)=w3849) -> (substring=w3848:string)  [unwired: 1 out]
                n940 = To Double Precision Float(number=w3836) -> (double precision float=w3835:dbl)
                n941 = Concatenate Strings(w3848, "_pos.dat" ("string")) -> (w3846:string)
                n942 = Build Array (concatenate)(w3835, w3834) -> (w3832:dbl[])
                n943 = String To Path(string=w3846) -> (path=w3842:path)
                n944 = Open/Create/Replace File(file path (use dialog)=w3842, operation (0:open)=T37."create", access (0:read/write)=enum16{"read/write", "read-only", "write-only"}."write-only") -> (refnum out=w3843:refnum<file>)  [unwired: 1 in, 4 out]
                n945 = Deny Access(7:w3843) -> (3:w3839:refnum<file>)  [unwired: 1 in, 2 out]
                n946 = Write to Binary File(file (use dialog)=w3839, data=w3832, 5:FALSE ("prepend array or string size? (T)"), 9:T38."big-endian, network order" ("byte order (0:big-endian, network order)")) -> (refnum out=w3837:refnum<file>)  [unwired: 1 in, 3 out]
              }
            }
            n947 = Write to Binary File(file (use dialog)=w3823, data=w3808, 5:w3804, 9:w3802) -> (refnum out=w3805:refnum<file>)  [unwired: 1 in, 3 out]
            n948 = Write to Binary File(file (use dialog)=w3805, data="Comment (data description)", 5:w3804, 9:w3802) -> (refnum out=w3801:refnum<file>)  [unwired: 1 in, 3 out]
          }
        }
        n949 = feedback-in #19(w3744) -> ()
        n950 = feedback-in #20(w3771) -> ()
        n951 = feedback-in #21(w3743) -> ()
        n952 = feedback-in #22(w3754) -> ()
        n953 = feedback-in #23(w3757) -> ()
        n954 = feedback-in #24(w3770) -> ()
        n955 = feedback-in #25(w3760) -> ()
      }
      frame #1 {
        n956 = local read "Saving..."() -> (w4001:bool)
        n957 = case shown="True" w4001 {
          tunnel: w4005 -> [_ w4015]
          tunnel: w4004 -> [_ w4029]
          tunnel: w4003 -> [_ w4025]
          tunnel: w4002 -> [_ w4024]
          tunnel: w4000 -> [_ w4023]
          tunnel: w3999 -> [_ w4018]
          tunnel: w3998 -> [_ w4017]
          tunnel: w3997 -> [_ w4016]
          tunnel: w3996 -> [_ w4014]
          tunnel: w3995 -> [_ w4012]
          tunnel: w3994 -> [_ w4011]
          tunnel: w3993 -> [_ w4010]
          tunnel: w3992 -> [_ w4009]
          tunnel: w3991 -> [_ w4008]
          tunnel: w3990 -> [_ w4007]
          tunnel: w3989 -> [_ w4006]
          frame False {
          }
          frame True {
            n958 = Multiply(x=w4015, y=w4014) -> (x*y=→"Time (s)":dbl)
            n959 = Less Or Equal?(x=w4015, y=w4023) -> (x <= y?=w4027:bool)
            n960 = Or(x="Stop Saving", y="Abort save 2") -> (x .or. y?=w4019:bool)
            n961 = Not(x=w4019) -> (.not. x?=w4028:bool)
            n962 = And(x=w4027, y=w4028) -> (x .and. y?=w4026:bool)
            n963 = case shown="True" w4026 {
              tunnel: w4029 -> [w4036 w4104]
              tunnel: [0.0 w4107] -> w4022
              tunnel: w4015 -> [_ w4105]
              tunnel: w4023 -> [_ w4106]
              tunnel: w4025 -> [_ w4101]
              tunnel: w4024 -> [_ _]
              tunnel: w4018 -> [w4034 w4094]
              tunnel: w4017 -> [w4033 w4095]
              tunnel: w4016 -> [_ w4093]
              tunnel: w4012 -> [_ w4092]
              tunnel: w4011 -> [_ w4046]
              tunnel: w4010 -> [_ w4085]
              tunnel: w4009 -> [_ w4063]
              tunnel: w4008 -> [w4030 w4044]
              tunnel: w4007 -> [w4031 w4043]
              tunnel: w4006 -> [_ w4040]
              frame False {
                w4032 = FALSE
                n964 = Close File(refnum=w4036) -> ()  [unwired: 1 in, 2 out]
                n965 = case shown="True" w4033 {
                  tunnel: w4034 -> [_ w4038]
                  frame False {
                  }
                  frame True {
                    n966 = Close File(refnum=w4038) -> ()  [unwired: 1 in, 2 out]
                  }
                }
                n967 = case shown="True" w4030 {
                  tunnel: w4031 -> [_ w4037]
                  frame False {
                  }
                  frame True {
                    n968 = Close File(refnum=w4037) -> ()  [unwired: 1 in, 2 out]
                  }
                }
                n969 = local write "Raster Scanning..."(w4032) -> ()
                n970 = local write "Calibrating Trap..."(w4032) -> ()
                n971 = call <vilib>:"Beep.vi"() -> ()  [unwired: 3 in, 9 out]
                n972 = local write "Stop Saving"(w4032) -> ()
                "Saving..." <- w4032
              }
              frame True {
                n973 = local read "Calibrating Trap..."() -> (w4096:bool)
                n974 = case "Write fl. data" shown="True" w4095 {
                  tunnel: w4094 -> [_ w4130]
                  tunnel: w4093 -> [_ w4129]
                  frame False {
                  }
                  frame True {
                    n975 = Write to Binary File(file (use dialog)=w4130, data=w4129, 5:FALSE ("prepend array or string size? (T)"), 9:T38."big-endian, network order" ("byte order (0:big-endian, network order)")) -> ()  [unwired: 1 in, 4 out]
                  }
                }
                n976 = Greater?(x="Save ave N", y=1.0) -> (0:w4099:bool)
                n977 = Not(x=w4096) -> (.not. x?=w4098:bool)
                n978 = And(x=w4098, y=w4099) -> (x .and. y?=w4041:bool)
                n979 = case shown="True" w4041 {
                  tunnel: w4040 -> [w4110 w4121]
                  tunnel: [w4110 w4113] -> w4039
                  tunnel: "Save ave N" -> [_ w4114]
                  frame False {
                  }
                  frame True {
                    w4111 = 2 ("dimension size")
                    n980 = Array Size(array=w4121) -> (size(s)=w4115:i32)
                    n981 = Divide(x=w4115, y=w4111) -> (x/y=w4119:dbl)
                    n982 = Reshape Array(w4121, w4119, w4111) -> (w4120:u64[][])
                    n983 = Transpose 2D Array(2D array=w4120) -> (transposed array=w4118:u64[][])
                    n984 = for {
                      tunnel: w4118 -> [w4123] mode=indexing
                      tunnel: [w4122] -> w4112 mode=indexing
                      tunnel: w4114 -> [w4124]
                      workers-P: _ -> [_]
                      n985 = call "downsample 1D array - U64.vi"("Ave N"=w4124, "Array In"=w4123) -> ("Array Out"=w4122:u64[])  [unwired: 1 in]
                    }
                    n986 = Transpose 2D Array(2D array=w4112) -> (transposed array=w4117:u64[][])
                    n987 = Divide(x=w4115, y=w4114) -> (x/y=w4116:dbl)
                    n988 = Reshape Array(w4117, w4116) -> (w4113:u64[])
                  }
                }
                n989 = case shown="True" w4041 {
                  tunnel: w4101 -> [w4133 w4145]
                  tunnel: [w4133 w4137] -> w4097
                  tunnel: "Save ave N" -> [_ w4138]
                  tunnel: w4092 -> [_ w4136]
                  frame False {
                  }
                  frame True {
                    n990 = Array Size(array=w4145) -> (size(s)=w4139:i32)
                    n991 = Array Size(array=w4136) -> (size(s)=w4135:i32)
                    n992 = Divide(x=w4139, y=w4135) -> (x/y=w4143:dbl)
                    n993 = Reshape Array(w4145, w4143, w4135) -> (w4144:i16[][])
                    n994 = Transpose 2D Array(2D array=w4144) -> (transposed array=w4142:i16[][])
                    n995 = for {
                      tunnel: w4142 -> [w4148] mode=indexing
                      tunnel: [w4147] -> w4134 mode=indexing
                      tunnel: w4138 -> [w4146]
                      workers-P: _ -> [_]
                      n996 = call "downsample 1D array - I16.vi"("Ave N"=w4146, "Array In"=w4148) -> ("Array Out"=w4147:i16[])  [unwired: 1 out]
                    }
                    n997 = Transpose 2D Array(2D array=w4134) -> (transposed array=w4141:i16[][])
                    n998 = Divide(x=w4139, y=w4138) -> (x/y=w4140:dbl)
                    n999 = Reshape Array(w4141, w4140) -> (w4137:i16[])
                  }
                }
                n1000 = Index Array(array=w4063, index=1) -> (element=w4066:waveform(dbl))
                n1001 = Index Array(array=w4063, index=0) -> (element=w4068:waveform(dbl))
                n1002 = Unbundle By Name(w4066) -> ("Y"=w4070:dbl[])
                n1003 = Unbundle By Name(w4068) -> ("Y"=w4078:dbl[])
                n1004 = case "Write trap pos. data" shown="True" w4044 {
                  tunnel: w4043 -> [_ w4126]
                  tunnel: w4039 -> [_ w4125]
                  frame False {
                  }
                  frame True {
                    n1005 = Write to Binary File(file (use dialog)=w4126, data=w4125, 5:FALSE ("prepend array or string size? (T)"), 9:T38."big-endian, network order" ("byte order (0:big-endian, network order)")) -> ()  [unwired: 1 in, 4 out]
                  }
                }
                n1006 = Write to Binary File(file (use dialog)=w4104, data=w4097, 5:FALSE ("prepend array or string size? (T)"), 9:T38."big-endian, network order" ("byte order (0:big-endian, network order)")) -> ()  [unwired: 1 in, 4 out]
                n1007 = feedback #26(w4070) -> (w4072:dbl[])
                n1008 = Build Array (concatenate)(w4072, w4070) -> (w4071:dbl[])
                n1009 = Select(t=w4070, s=w4046, f=w4071) -> (s? t:f=w4056:dbl[])
                n1010 = feedback-in #26(w4056) -> ()
                n1011 = feedback #27(w4078) -> (w4091:dbl[])
                n1012 = Build Array (concatenate)(w4091, w4078) -> (w4090:dbl[])
                n1013 = Select(t=w4078, s=w4046, f=w4090) -> (s? t:f=w4065:dbl[])
                n1014 = feedback-in #27(w4065) -> ()
                n1015 = Divide(x=w4105, y=w4106) -> (x/y=w4108:dbl)
                n1016 = Multiply(x=w4108, y=100.0) -> (x*y=w4107:dbl)
                n1017 = Build Array(w4065, w4056) -> (→"Saved APD":dbl[][])
                n1018 = Array Size(array=w4065) -> (size(s)=w4083:i32)
                n1019 = Unbundle By Name(w4085) -> ("Y"=w4089:dbl[])
                n1020 = Subtract(x=w4083, y="N pts to average") -> (x-y=w4059:i32)
                n1021 = Multiply(x="N pts to average", y=u16 2) -> (x*y=w4060:u16)
                n1022 = Subtract(x=w4083, y=w4060) -> (x-y=w4058:i32)
                n1023 = feedback #28(w4089) -> (w4088:dbl[])
                n1024 = Build Array (concatenate)(w4088, w4089) -> (w4087:dbl[])
                n1025 = Select(t=w4089, s=w4046, f=w4087) -> (s? t:f=w4086:dbl[])
                "Trap Delta Graph" <- w4086
                n1026 = feedback-in #28(w4086) -> ()
                n1027 = Array Subset(array=w4065, index=w4059, length="N pts to average") -> (w4082:dbl[])
                n1028 = Array Subset(array=w4065, index=w4058, length="N pts to average") -> (w4081:dbl[])
                n1029 = Array Subset(array=w4056, index=w4059, length="N pts to average") -> (w4062:dbl[])
                n1030 = Array Subset(array=w4056, index=w4058, length="N pts to average") -> (w4061:dbl[])
                n1031 = call <vilib>:"Mean.vi"("X"=w4082) -> ("mean"=w4080:dbl)  [unwired: 1 out]
                n1032 = call <vilib>:"Mean.vi"("X"=w4062) -> ("mean"=w4055:dbl)  [unwired: 1 out]
                n1033 = call <vilib>:"Mean.vi"("X"=w4081) -> ("mean"=w4079:dbl)  [unwired: 1 out]
                n1034 = call <vilib>:"Mean.vi"("X"=w4061) -> ("mean"=w4054:dbl)  [unwired: 1 out]
                n1035 = Subtract(x=w4055, y=w4054) -> (x-y=w4045:dbl)
                "Delta Fl. 2" <- w4045
                n1036 = Subtract(x=w4080, y=w4079) -> (x-y=w4077:dbl)
                "Delta Fl. 1" <- w4077
                n1037 = Initialize Array(w4077, 1 ("dimension size")) -> (w4074:dbl[])
                n1038 = Initialize Array(w4045, 1 ("dimension size")) -> (w4051:dbl[])
                n1039 = feedback #29(w4074) -> (w4075:dbl[])
                n1040 = Build Array (concatenate)(w4075, w4074) -> (w4073:dbl[])
                n1041 = feedback #30(w4051) -> (w4052:dbl[])
                n1042 = Build Array (concatenate)(w4052, w4051) -> (w4050:dbl[])
                n1043 = Select(t=w4074, s=w4046, f=w4073) -> (s? t:f=w4049:dbl[])
                n1044 = feedback-in #29(w4049) -> ()
                n1045 = Select(t=w4051, s=w4046, f=w4050) -> (s? t:f=w4048:dbl[])
                n1046 = feedback-in #30(w4048) -> ()
                n1047 = Build Array(w4049, w4048) -> (→"Save APD Deriv":dbl[][])
              }
            }
            "Progress" <- w4022
            "Progress 2" <- w4022
          }
        }
      }
    }
    n1048 = Bundle By Name(cluster=w1131, "Green FB Ch 0"=w1130, "Green FB Ch 1"=w1129) -> (w1109:T45)
    "Green FB Signals (V)" <- w1109
    n1049 = Unbundle By Name(w1109) -> ("Green FB Ch 2"=→"Green FB Plot":dbl)
    n1050 = local read "wait to reset values"() -> (w1201:bool)
    n1051 = Not(x=w1198) -> (.not. x?=w1202:bool)
    n1052 = And(x=w1202, y=w1201) -> (x .and. y?=w1203:bool)
    n1053 = case "Part of MCL raster scanning: returns to initial positions after scan done" shown="True" w1203 {
      tunnel: w1206 -> [w2739 w2746]
      tunnel: [w2739 w2745] -> w1205
      tunnel: w1200 -> [w2738 w2744]
      tunnel: [w2738 w2743] -> w1199
      frame False {
      }
      frame True {
        w2754 = 10.0 ("y")
        w2753 = 32767.0 ("y")
        # "to return scan values\nafter a synchronous \nAOM scan"
        n1054 = local read "AO2"() -> (w2747:dbl)
        n1055 = local read "AO1"() -> (w2748:dbl)
        n1056 = local write "wait to reset values"(FALSE ("wait to reset values")) -> ()
        n1057 = Multiply(x=w2748, y=w2753) -> (x*y=w2750:dbl)
        n1058 = Multiply(x=w2747, y=w2753) -> (x*y=w2752:dbl)
        n1059 = Divide(x=w2750, y=w2754) -> (x/y=w2749:dbl)
        n1060 = Divide(x=w2752, y=w2754) -> (x/y=w2751:dbl)
        n1061 = To Word Integer(number=w2749) -> (16bit integer=w2755:i16)
        n1062 = To Word Integer(number=w2751) -> (16bit integer=w2756:i16)
        n1063 = local read "Total Counts (ticks)"() -> (w2740:u32)
        n1064 = xnode "Read/Write Control"("FPGA VI Reference In"=w2746, "error in"=w2744, "AO1"=w2755, "AO2"=w2756, "MCL count"=w2740) -> ("FPGA VI Reference Out"=w2745:T20, "error out"=w2743:errorcluster)